vi "ScanDelay_FTIR.vi"() -> ()   [LabVIEW 2021]
uses:
  ScanDelay/Control_scanDelayWorkflow.ctl
  C:/Users/mnopl/Desktop/Software/LabVIEW/PRISM Scanning/Thorlabs.MotionControl.Controls.dll
  Thorlabs.MotionControl.Controls.dll
panel:
  in  "Cancel\nacquisition":bool
  in  "SerialNumber Flipper":string="37005305"
  in  "FilterFlipperControl":refnum<k24>(container)
  out "Spectrum stored":bool=TRUE
  out "Reference stored":bool=TRUE
  out "Normalized spectrum (phase)":T1(graph)={"Output spectrum"=[1102.5289175333148, 1103.2115979776079, 1103.894278421901, 1104.576958866194, 1105.259639310487, 1105.94231975478, 1106.6250001990732, 1107.3076806433662, 1107.9903610876595, 1108.6730415319525, 1109.3557219762456, 1110.0384024205387, 1110.7210828648317, 1111.4037633091248, 1112.0864437534178, 1112.7691241977109, 1113.451804642004, 1114.134485086297, 1114.81716553059, 1115.499845974883, 1116.1825264191764, 1116.8652068634694, 1117.5478873077625, 1118.2305677520555, 1118.9132481963486, 1119.5959286406417, 1120.2786090849347, 1120.9612895292278, 1121.6439699735208, 1122.3266504178139, 1123.009330862107, 1123.6920113064, 1124.3746917506933, 1125.0573721949863, 1125.7400526392794, 1126.4227330835724, 1127.1054135278655, 1127.7880939721585, 1128.4707744164516, 1129.1534548607447, 1129.8361353050377, 1130.5188157493308, 1131.2014961936238, 1131.8841766379169, 1132.5668570822102, 1133.2495375265032, 1133.9322179707963, 1134.6148984150893, 1135.2975788593824, 1135.9802593036754, 1136.6629397479685, 1137.3456201922615, 1138.0283006365546, 1138.7109810808477, 1139.3936615251407, 1140.0763419694338, 1140.759022413727, 1141.44170285802, 1142.1243833023132, 1142.8070637466062, 1143.4897441908993, 1144.1724246351923, 1144.8551050794854, 1145.5377855237784, 1146.2204659680715, 1146.9031464123645, 1147.5858268566576, 1148.2685073009507, 1148.951187745244, 1149.633868189537, 1150.31654863383, 1150.999229078123, 1151.6819095224162, 1152.3645899667092, 1153.0472704110023, 1153.7299508552953, 1154.4126312995884, 1155.0953117438814, 1155.7779921881745, 1156.4606726324675, 1157.1433530767608, 1157.826033521054, 1158.508713965347, 1159.19139440964, 1159.874074853933, 1160.556755298226, 1161.2394357425192, 1161.9221161868122, 1162.6047966311053, 1163.2874770753983, 1163.9701575196914, 1164.6528379639844, 1165.3355184082777, 1166.0181988525708, 1166.7008792968638, 1167.383559741157, 1168.06624018545, 1168.748920629743, 1169.431601074036, 1170.114281518329, 1170.7969619626222, 1171.4796424069152, 1172.1623228512083, 1172.8450032955013, 1173.5276837397946, 1174.2103641840877, 1174.8930446283807, 1175.5757250726738, 1176.2584055169668, 1176.94108596126], "Output spectrum"=[-1.328981625574806, -1.3297156380454427, -1.332925494608056, -1.3383669398670515, -1.3490986679786652, -1.3620665887791494, -1.3728322840821798, -1.3808051789599451, -1.38268785735066, -1.383454007683691, -1.3867362370563832, -1.392628994922722, -1.4079022417461098, -1.4232661538457454, -1.4254793325337713, -1.4234088794856259, -1.4261421511209245, -1.4345438849308945, -1.450738970302403, -1.4651556417192133, -1.472033577259217, -1.4765650658678406, -1.4767899466709609, -1.4779591915412682, -1.4864306235316898, -1.4967145833357045, -1.509311752447231, -1.5200946146126175, -1.5203325079241412, -1.518823068339795, -1.5221051369918865, -1.5289919543416084, -1.5443021693708103, -1.5596522358123068, -1.564563007819482, -1.564695009899656, -1.563485351619463, -1.564979237220899, -1.575817473163252, -1.5890558529666865, -1.598676891266045, -1.6047391447914532, -1.6037521530971257, -1.6021261032252092, -1.6080019905637195, -1.6176268726411671, -1.6308671920818638, -1.6420882814095819, -1.641366971284346, -1.6377105789186341, -1.6370525992687766, -1.6391413606802254, -1.6515063645518546, -1.6657201783289788, -1.6701214238463176, -1.6692686137411459, -1.664673373679217, -1.662735930327408, -1.6725089834242368, -1.6846208268448783, -1.6936098642043782, -1.6989794868515014, -1.6946893180335745, -1.6887570609947458, -1.6897142609229832, -1.6962784013144874, -1.7104316701396314, -1.7219554489591749, -1.7205768313097645, -1.716071748236028, -1.7122923695362096, -1.71258756824989, -1.7254368375091567, -1.7398505346411333, -1.74608798471659, -1.7471789380119624, -1.740606874293851, -1.7349037247161565, -1.7402490589291773, -1.7516392441731288, -1.7671122393723413, -1.7758636915304795, -1.7693645101770739, -1.7643499082781715, -1.7637118229070248, -1.765350147635751, -1.7796219339063313, -1.7937296960608236, -1.7953854575566122, -1.7914716614824544, -1.7856026813204544, -1.784818380975335, -1.7962387728445355, -1.812386692062692, -1.8233317957340986, -1.8247979168699975, -1.8161391987680926, -1.8112956667262592, -1.8161667026018287, -1.8247366793368631, -1.8389102094421166, -1.8495163568361097, -1.8449801698590533, -1.8376790464210524, -1.8356629006103997, -1.8413241156179243, -1.860416535366724, -1.8782177477731439, -1.881203280417375, -1.8755210713733286]}
  out "Normalized spectrum (amplitude)":T1(graph)={"Output spectrum"=[1102.5289175333148, 1103.2115979776079, 1103.894278421901, 1104.576958866194, 1105.259639310487, 1105.94231975478, 1106.6250001990732, 1107.3076806433662, 1107.9903610876595, 1108.6730415319525, 1109.3557219762456, 1110.0384024205387, 1110.7210828648317, 1111.4037633091248, 1112.0864437534178, 1112.7691241977109, 1113.451804642004, 1114.134485086297, 1114.81716553059, 1115.499845974883, 1116.1825264191764, 1116.8652068634694, 1117.5478873077625, 1118.2305677520555, 1118.9132481963486, 1119.5959286406417, 1120.2786090849347, 1120.9612895292278, 1121.6439699735208, 1122.3266504178139, 1123.009330862107, 1123.6920113064, 1124.3746917506933, 1125.0573721949863, 1125.7400526392794, 1126.4227330835724, 1127.1054135278655, 1127.7880939721585, 1128.4707744164516, 1129.1534548607447, 1129.8361353050377, 1130.5188157493308, 1131.2014961936238, 1131.8841766379169, 1132.5668570822102, 1133.2495375265032, 1133.9322179707963, 1134.6148984150893, 1135.2975788593824, 1135.9802593036754, 1136.6629397479685, 1137.3456201922615, 1138.0283006365546, 1138.7109810808477, 1139.3936615251407, 1140.0763419694338, 1140.759022413727, 1141.44170285802, 1142.1243833023132, 1142.8070637466062, 1143.4897441908993, 1144.1724246351923, 1144.8551050794854, 1145.5377855237784, 1146.2204659680715, 1146.9031464123645, 1147.5858268566576, 1148.2685073009507, 1148.951187745244, 1149.633868189537, 1150.31654863383, 1150.999229078123, 1151.6819095224162, 1152.3645899667092, 1153.0472704110023, 1153.7299508552953, 1154.4126312995884, 1155.0953117438814, 1155.7779921881745, 1156.4606726324675, 1157.1433530767608, 1157.826033521054, 1158.508713965347, 1159.19139440964, 1159.874074853933, 1160.556755298226, 1161.2394357425192, 1161.9221161868122, 1162.6047966311053, 1163.2874770753983, 1163.9701575196914, 1164.6528379639844, 1165.3355184082777, 1166.0181988525708, 1166.7008792968638, 1167.383559741157, 1168.06624018545, 1168.748920629743, 1169.431601074036, 1170.114281518329, 1170.7969619626222, 1171.4796424069152, 1172.1623228512083, 1172.8450032955013, 1173.5276837397946, 1174.2103641840877, 1174.8930446283807, 1175.5757250726738, 1176.2584055169668, 1176.94108596126], "Output spectrum"=[1.0873076708633411, 1.08394867428729, 1.0888562107920463, 1.0969307314805181, 1.102998120422263, 1.107136071600766, 1.1035642445072202, 1.0961034542227839, 1.094872735773217, 1.1010416062836017, 1.1106100405553267, 1.115942213485196, 1.1130278245062957, 1.1072973234979273, 1.102059722167887, 1.098186618808356, 1.1015816281752067, 1.108746473864395, 1.111756741956775, 1.1105953151312484, 1.1032227061156759, 1.0952300942782656, 1.0958494687443006, 1.1007057231621713, 1.106295224941442, 1.1104780174250957, 1.1057667534821705, 1.0964576694777417, 1.0904090869006036, 1.088459311408212, 1.0942598558444103, 1.1012239259596472, 1.0993344675621843, 1.092466822796523, 1.0835822296721949, 1.0759964933630453, 1.0774338793339753, 1.0829818692266655, 1.085123774157756, 1.0835731005973663, 1.0747228497785382, 1.0629565097932145, 1.0579906286730316, 1.058422967601046, 1.0630212715521237, 1.0675638836007573, 1.0625734863702079, 1.0529318841119182, 1.0449994916681102, 1.0391477625279653, 1.0421567088004438, 1.0486532412237262, 1.0477398261213626, 1.0417732985786687, 1.03113814399867, 1.0200979633688834, 1.0182230978827198, 1.022584163574115, 1.0286739828363953, 1.032026518895644, 1.0242044127425998, 1.011323536655613, 1.0049354451214019, 1.0053102459549301, 1.011993306853234, 1.0193524696815321, 1.0176245623256048, 1.0098015162659275, 0.9995985179330682, 0.9919293607652324, 0.995810871440088, 1.0045616890791953, 1.0093618831764462, 1.008860094407166, 0.9990320036845148, 0.9874622731652223, 0.9856201758039206, 0.9912449764462133, 0.9997370337275218, 1.0041657589490753, 0.9979424163566785, 0.9878008483696279, 0.9797038935662515, 0.9774024796092163, 0.9873954031846796, 0.9975940631540408, 0.996754666997269, 0.990809571391422, 0.9797449519284779, 0.9700271866511746, 0.9728145275232338, 0.9828560719840351, 0.9916163639682382, 0.9946994569688331, 0.9866468392828865, 0.9740403779039128, 0.9670830091995587, 0.9689347920073221, 0.9807941187046116, 0.9896212414408725, 0.9843156725932524, 0.9762091225257215, 0.969940310795789, 0.9659022733566544, 0.9737200015171775, 0.9861338055781489, 0.988751689371605, 0.983147618233142, 0.9731806985492104, 0.9653668962641432]}
  in  "Store as reference":bool
  out "Python alpha rep path":path=path "C:/Users/mnopl/Desktop/Software/python/alpha/rep.py"
  out "Activity status":string="Awaiting command"
  out "Acquisition status":string="Ready to acquire spectrum"
  in  "Save spectrum to path":path
  in  "Load reference":bool
  in  "Load reference from path":path
  in  "Load spectrum from path":path
  in  "Apply spectral\nenvelope":bool=TRUE
  out "Binned interferogram":cluster{"X":dbl, "Y":dbl}[](graph)
  out "Reference Spectra":dbl[][](array[numeric])
  out "Analyte Spectra":dbl[][](array[numeric])
  out "Python error: spectrum acquisition":errorcluster={"status"=TRUE, "code"=1666, "source"="Python Node in ScanDelay_FTIR.vi"}
  out "Python scandelay path":path=path "C:/Users/mnopl/Desktop/Software/LabVIEW/ScanDelay/scandelay.py"
  in  "Time per\nacquisition (s)":dbl=8.5
  in  "Sampling rate":dbl=250000.0
  in  "Delay calibration\n          factor":dbl=2.403 format="%_6g"
  in  "Acquisitions per\ninterferogram":i32=1
  in  "Bins per\ninterferogram":i32=30000
  in  "Subtract\nphase slope\n (2pi * dx)":dbl=-0.001
  out "Python error: DAQ acquisition":errorcluster
  out "# Accumulated":i32=4
  in  "Accumulate to #":i32=4
  out "Latest alpha cmd":string="@rep load 9"
  in  "Replicate alpha\non accumulate?":bool
  out "Accumulated spectrum (amplitude)":T1(graph)
  out "Accumulated spectrum (phase)":T1(graph)
  out "Acquisition cycle":dbl[][](graph)
  out "% averaged":dbl=100.0
  in  "Pause\nacquisition":bool
  in  "Halt program":bool
  out "Python error: activity loop":errorcluster
  in  "Load spectrum":bool
  in  "Save spectrum":bool
  in  "Normalize spectrum":bool
  in  "Acquire spectrum":bool
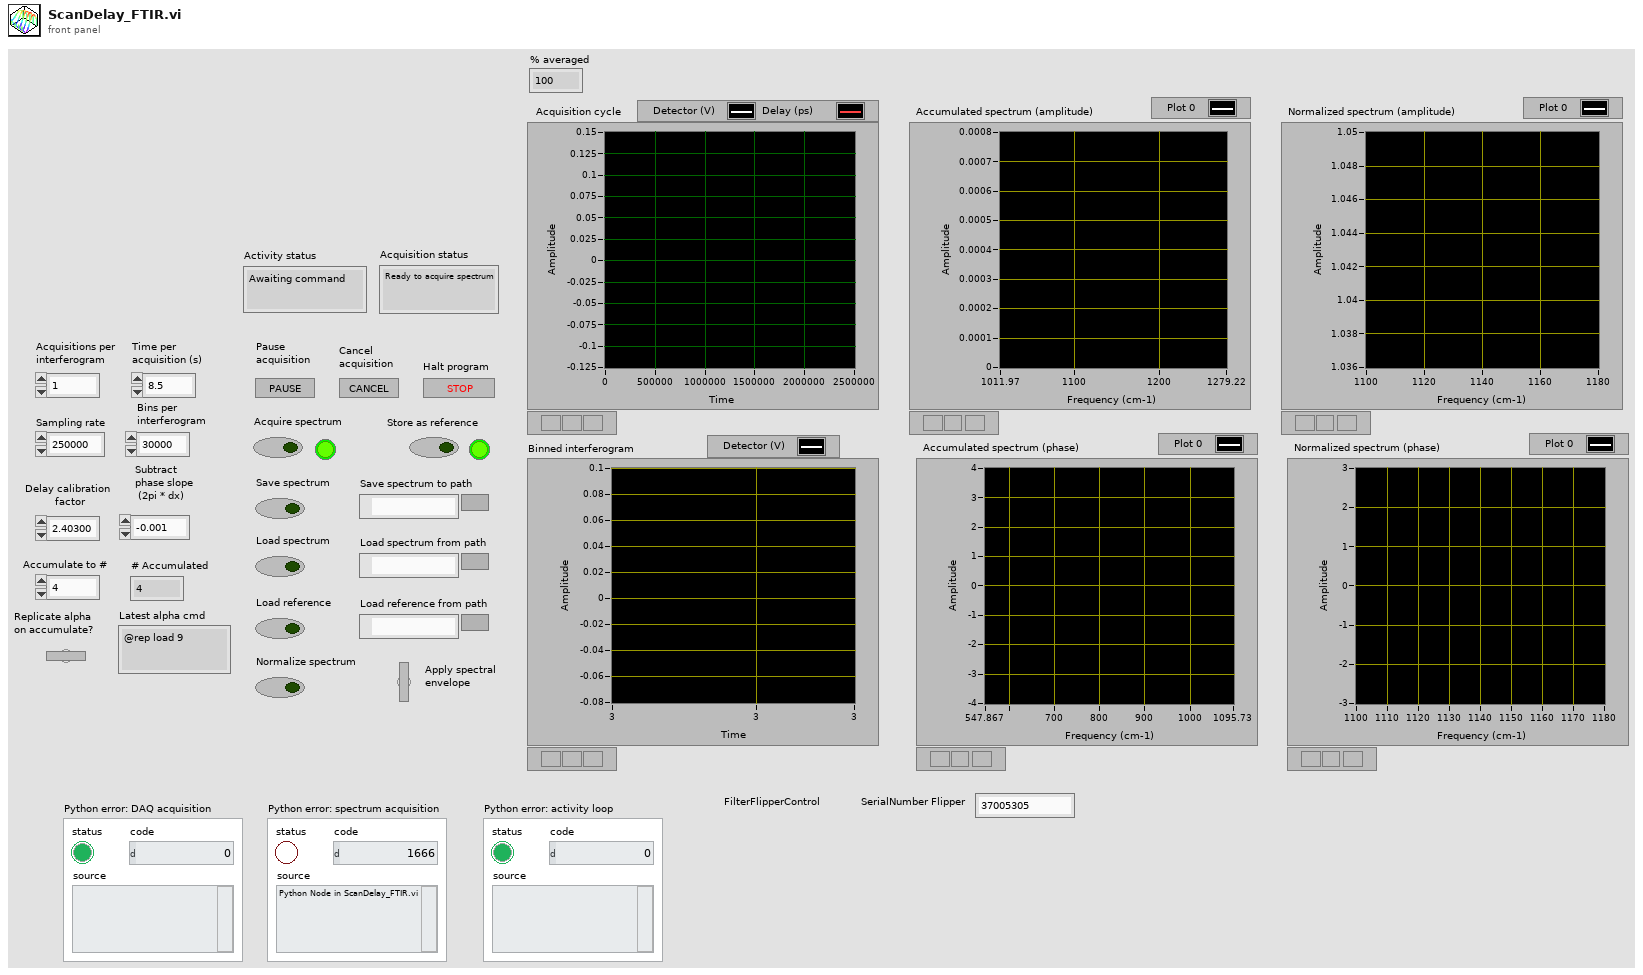
[diagram p1: front panel]
types:
  T1 = cluster{"Output spectrum":dbl[], "Output spectrum":dbl[]}
  T2 = typedef "Control_scanDelayWorkflow.ctl" = enum16{"Initialize", "Sit Idle", "Load Spectrum", "Store reference", "Save Spectrum", "Load reference", "Check Reference", "Check Spectrum", "Normalize Spectrum", "Done"}
  T3 = cluster{"Analyte Spectra":dbl[], "Analyte Spectra":dbl[]}
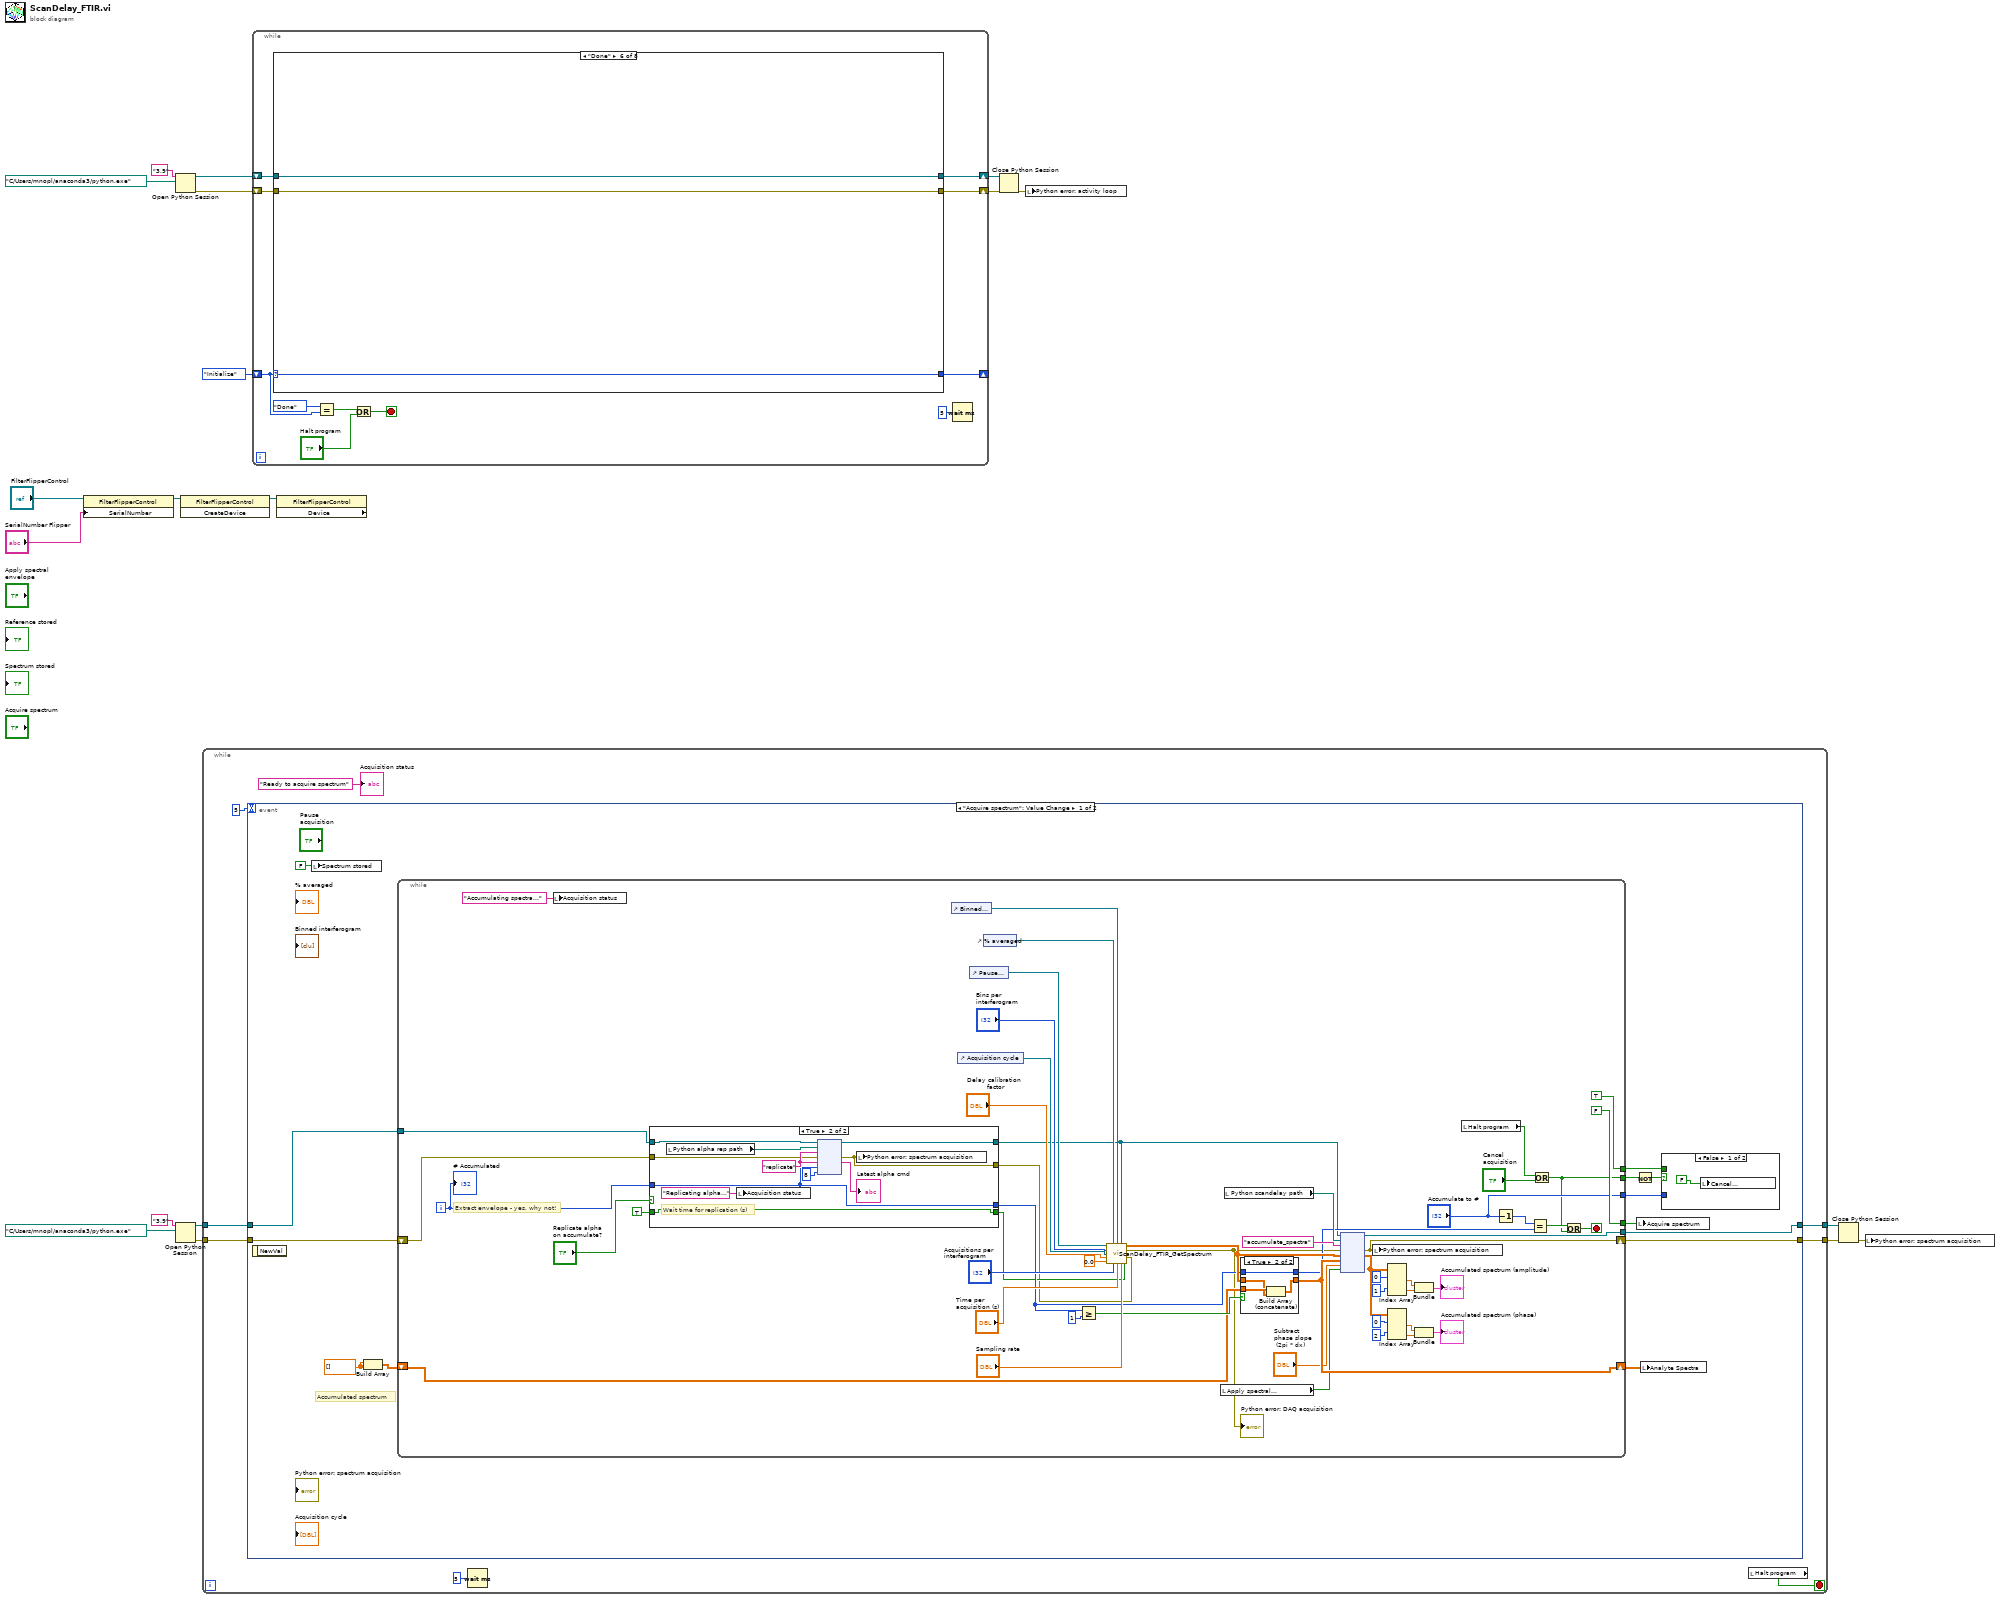
[diagram p0: block diagram]
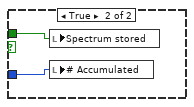
[diagram p2: hidden frame]
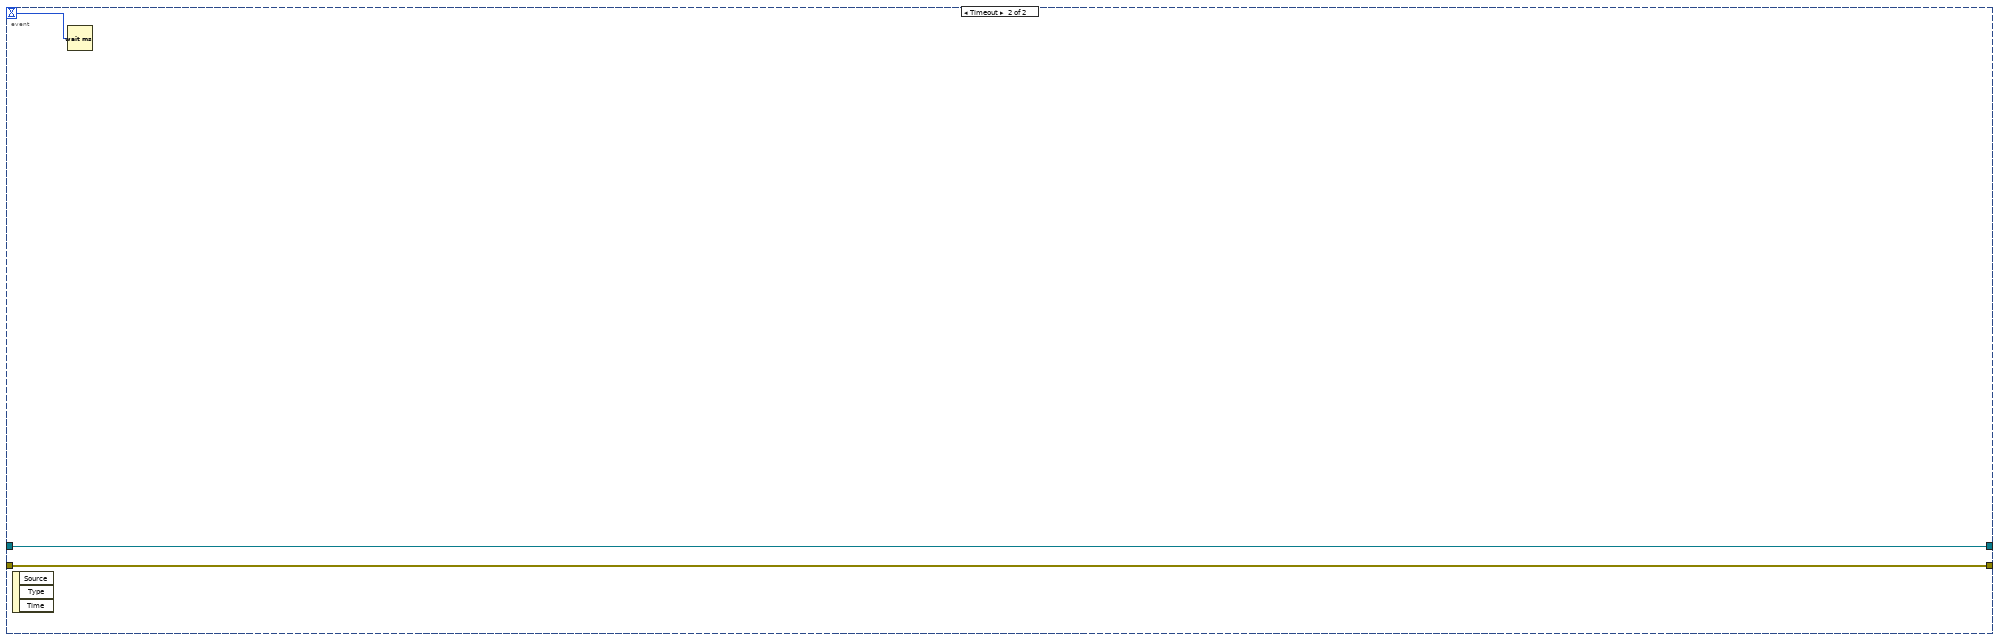
[diagram p5: hidden frame]
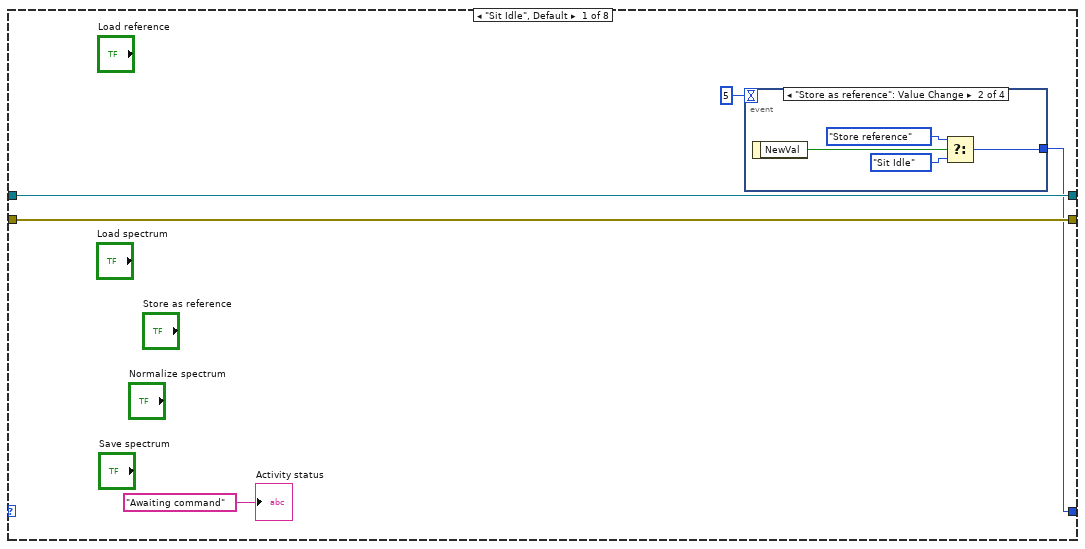
[diagram p6: hidden frame]
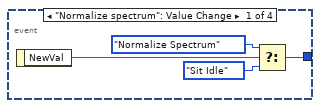
[diagram p7: hidden frame]
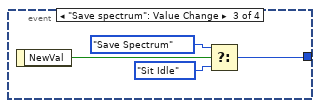
[diagram p8: hidden frame]
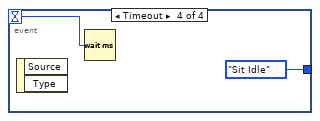
[diagram p9: hidden frame]
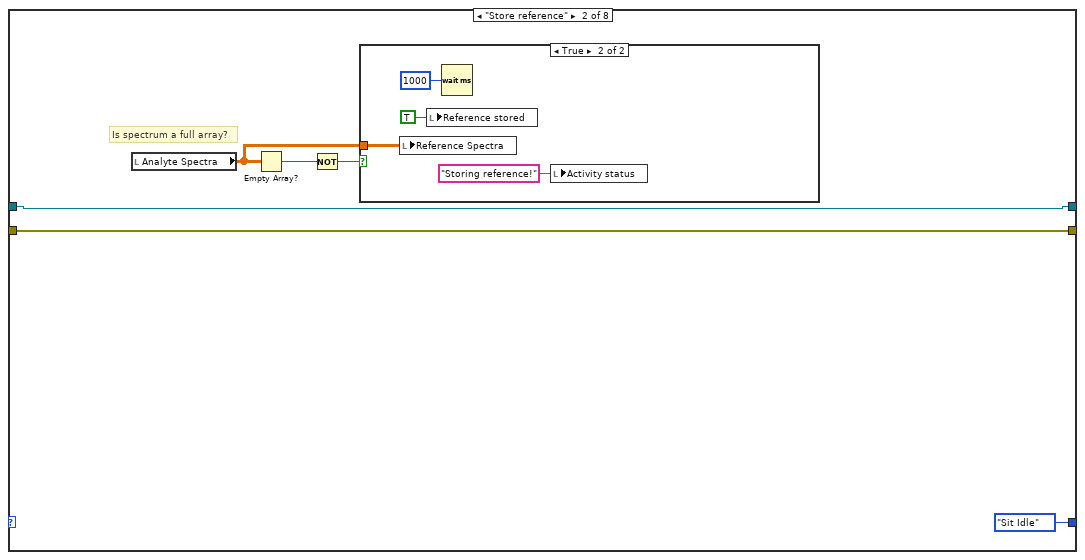
[diagram p10: hidden frame]
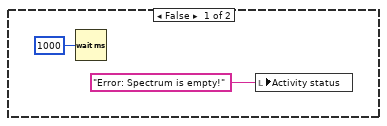
[diagram p11: hidden frame]
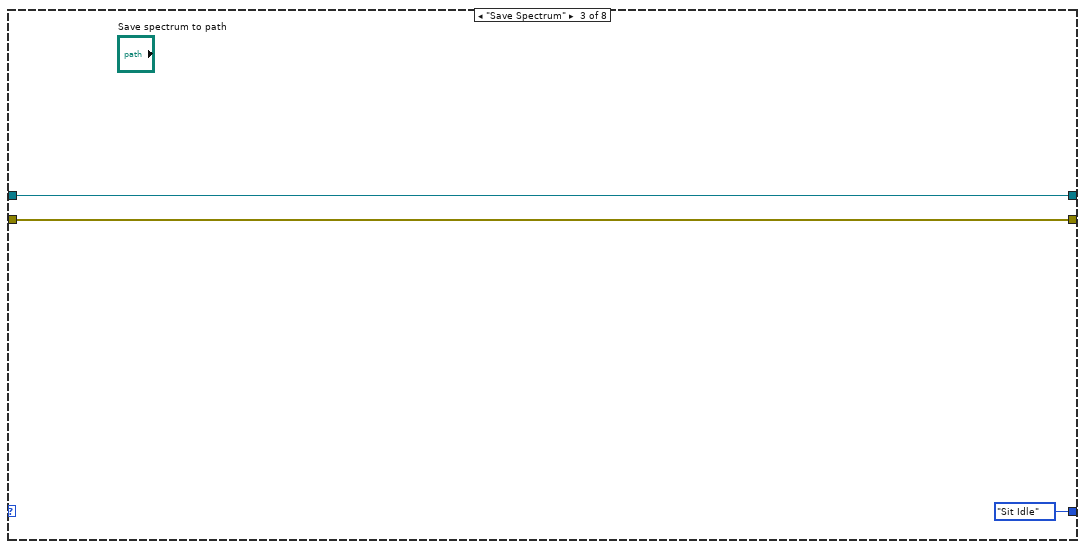
[diagram p12: hidden frame]
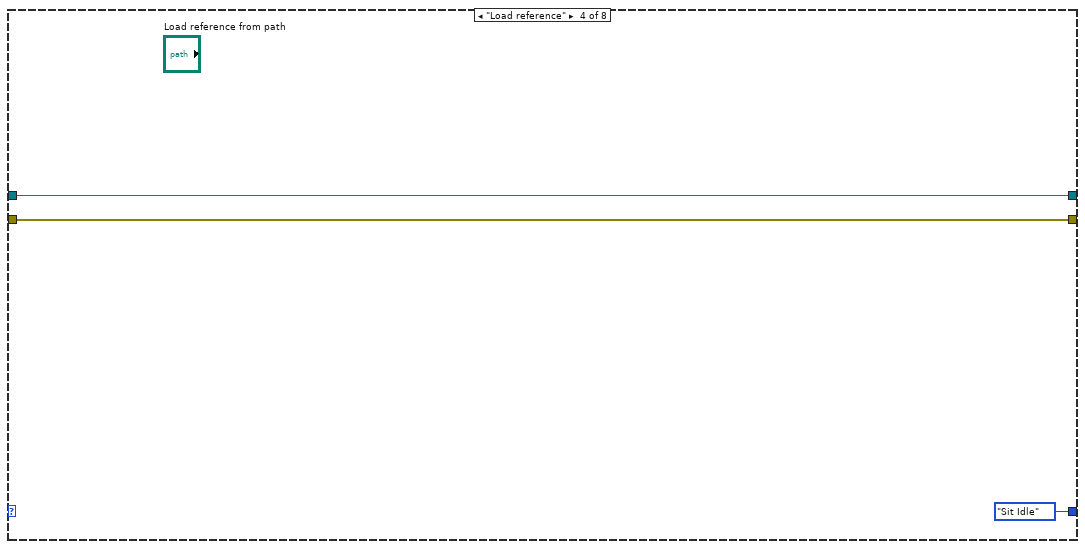
[diagram p13: hidden frame]
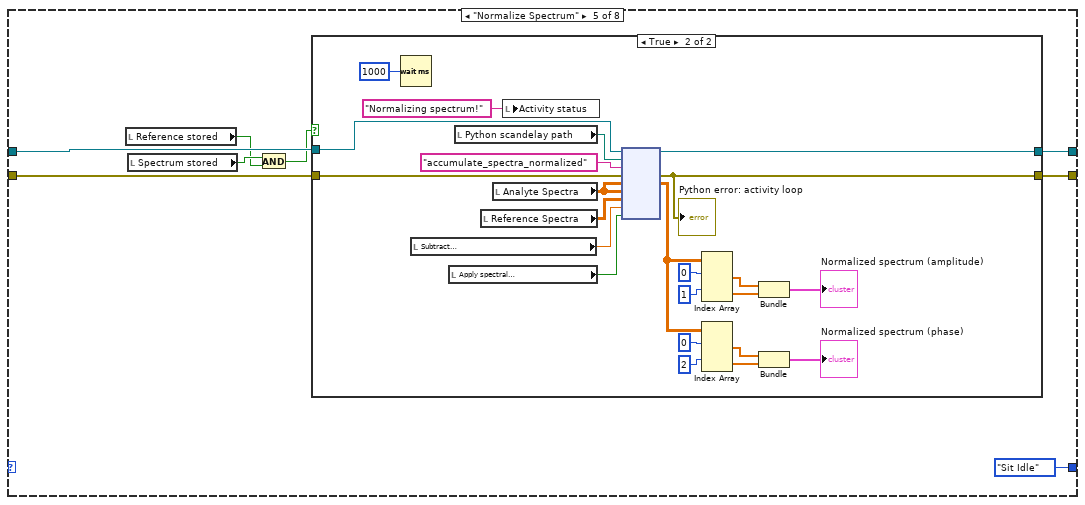
[diagram p14: hidden frame]
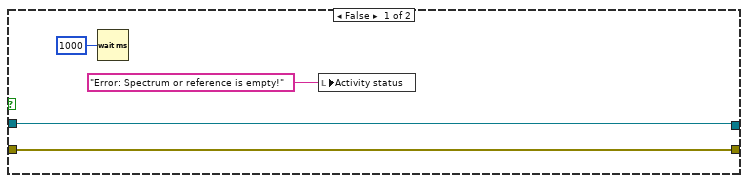
[diagram p15: hidden frame]
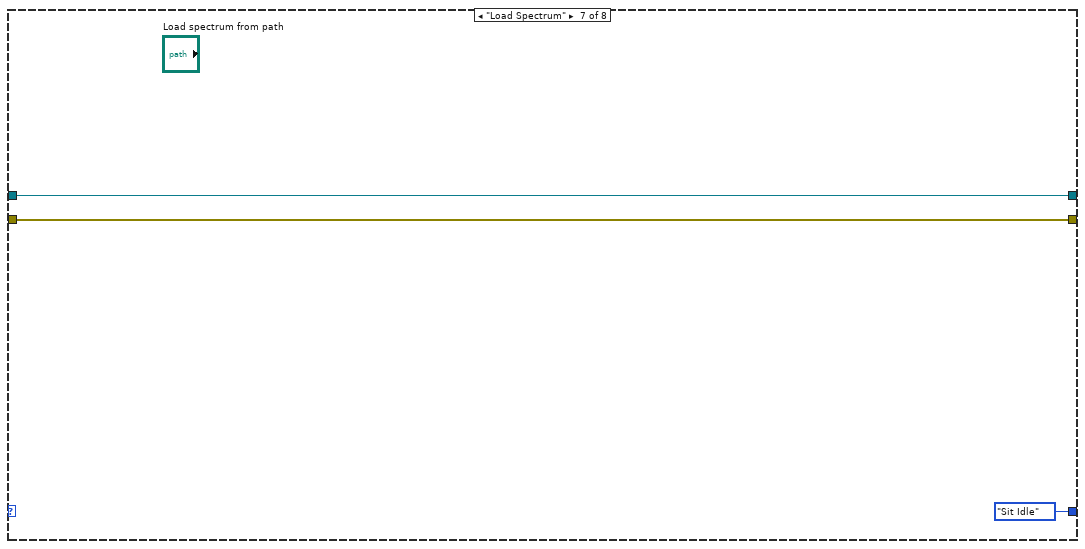
[diagram p16: hidden frame]
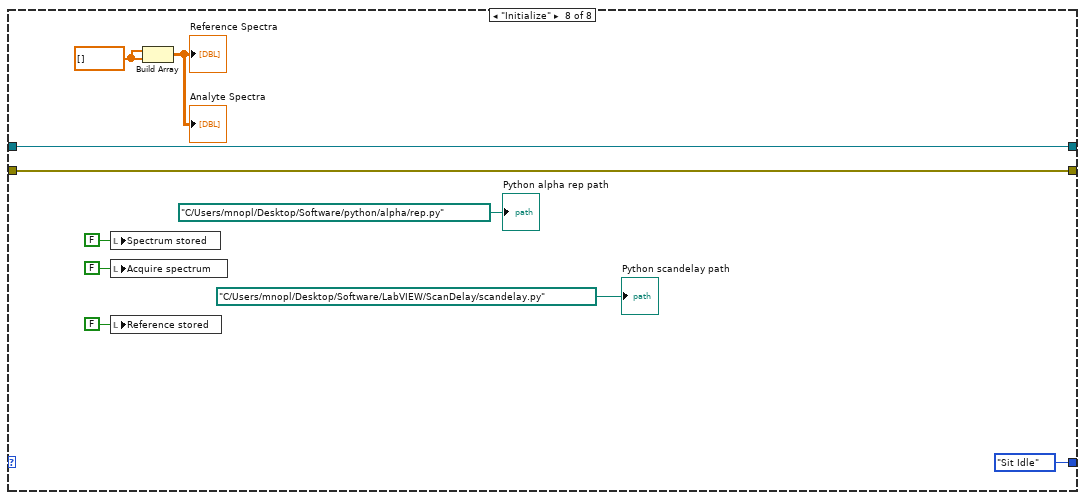
[diagram p17: hidden frame]
diagram:
  n1 = property class="FilterFlipperControl"(reference="FilterFlipperControl", "SerialNumber"="SerialNumber Flipper") -> (reference out=w2:refnum<k24>)  [unwired: 1 in, 1 out]
  n2 = Open Python Session(python version="3.9", python path=path "C:/Users/mnopl/anaconda3/python.exe") -> (session out=w8:refnum<k35>, error out=w7:errorcluster)  [unwired: 1 in]
  n3 = Open Python Session(python version="3.9", python path=path "C:/Users/mnopl/anaconda3/python.exe") -> (session out=w12:refnum<k35>, error out=w11:errorcluster)  [unwired: 1 in]
  n4 = invoke class="FilterFlipperControl" method="CreateDevice"(reference=w2) -> (reference out=w1:refnum<k24>)  [unwired: 2 in, 2 out]
  n5 = while {
    tunnel: w12 -> [w26]
    tunnel: w11 -> [w25]
    tunnel: [w24] -> w10
    tunnel: [w23] -> w9
    stop <- w27 stop-if-true
    n6 = event shown="[0] \"Acquire spectrum\": Value Change" {
      selector: _ -> [_ _]
      dyn-events: _ -> [_ _]
      timeout: 5 -> [_ w120]
      tunnel: w26 -> [w37 w118]
      tunnel: w25 -> [w36 w119]
      tunnel: [w35 w118] -> w24
      tunnel: [w33 w119] -> w23
      event "Acquire spectrum": Value Change {
        w39 = dbl[] []
        # "Accumulated spectrum"
        n7 = event-data() -> ()  [unwired: 1 in, 1 out]
        n8 = local write "Spectrum stored"(FALSE) -> ()
        n9 = Build Array(w39, w39) -> (w40:dbl[][])
        n10 = while {
          shift-right: [w74] -> w38
          shift-left: w40 -> [w87]
          tunnel: [w55] -> w35
          tunnel: w37 -> [w58]
          tunnel: [FALSE] -> w34
          shift-right: [w49] -> w33
          shift-left: w36 -> [w57]
          tunnel: [TRUE] -> w31
          tunnel: ["Accumulate to #"] -> w30
          tunnel: [w44] -> w28
          i -> [w51]
          stop <- w61 stop-if-true
          # "Extract envelope - yes, why not!"
          n11 = local write "Acquisition status"("Accumulating spectra...") -> ()
          n12 = case shown="True" "Replicate alpha\non accumulate?" {
            tunnel: w57 -> [w99 w108]
            tunnel: w58 -> [w100 w107]
            tunnel: [w100 w106] -> w46
            tunnel: [w99 w101] -> w48
            tunnel: w51 -> [w98 w103]
            tunnel: [w98 w103] -> w56
            tunnel: TRUE -> [w97 w102]
            tunnel: [w97 w102] -> w53
            frame False {
            }
            frame True {
              w109 = "replicate"
              # "Wait time for replication (s)"
              n13 = local read "Python alpha rep path"() -> (w104:path)
              n14 = local write "Acquisition status"("Replicating alpha...") -> ()
              n15 = node(w107, w104, w109, w108, w109, w103, 8) -> (w106:refnum<k35>, w101:errorcluster, →"Latest alpha cmd":string)  [unwired: 2 in, 2 out]
              n16 = local write "Python error: spectrum acquisition"(w101) -> ()
            }
          }
          n17 = control-ref of="Binned interferogram"() -> (w76:refnum<vi>)
          n18 = control-ref of="Acquisition cycle"() -> (w96:refnum<vi>)
          n19 = control-ref of="Pause\nacquisition"() -> (w91:refnum<vi>)
          n20 = control-ref of="% averaged"() -> (w92:refnum<vi>)
          n21 = Greater Or Equal?(x=w56, y=1) -> (x >= y?=w89:bool)
          n22 = call "ScanDelay_FTIR_GetSpectrum.vi"("Acquire / Pause? External"=w91, "% averaged (external)"=w92, "Binned interferogram (external)"=w76, "Python refnum in"=w46, "N delays"="Bins per\ninterferogram", "Acquisition cycle (external)"=w96, "Delay calibration\n          factor"="Delay calibration\n          factor", "Python error in"=w48, "Subtract\ndelay (ps)"=0.0, "Acquisitions per interferogram"="Acquisitions per\ninterferogram", "Time per acquisition (s)"="Time per\nacquisition (s)", "Sampling rate"="Sampling rate", "Extract envelope"=w53) -> ("Output spectrum"=w69:dbl[][], "Python error"=w47:errorcluster)  [unwired: 1 in]
          "Python error: DAQ acquisition" <- w47
          n23 = local read "Apply spectral\nenvelope"() -> (w65:bool)
          n24 = local read "Python scandelay path"() -> (w67:path)
          n25 = case shown="True" w89 {
            tunnel: w69 -> [w113 w116]
            tunnel: w87 -> [_ w117]
            tunnel: [w113 w115] -> w74
            tunnel: w56 -> [w112 w114]
            tunnel: [w112 w114] -> w52
            frame False {
            }
            frame True {
              n26 = Build Array (concatenate)(w117, w116) -> (w115:dbl[][])
            }
          }
          n27 = node(w46, w67, "accumulate_spectra", w47, w69, w74, "Subtract\nphase slope\n (2pi * dx)", w65) -> (w55:refnum<k35>, w49:errorcluster, w68:dbl[][])  [unwired: 3 in, 2 out]
          n28 = local write "Python error: spectrum acquisition"(w49) -> ()
          n29 = Index Array(array=w68, index (row) #1=0, index (row) #2=1) -> (element #1=w83:dbl[], element #2=w82:dbl[])  [unwired: 2 in]
          n30 = Index Array(array=w68, index (row) #1=0, index (row) #2=2) -> (element #1=w79:dbl[], element #2=w78:dbl[])  [unwired: 2 in]
          n31 = Bundle("Output spectrum"=w83, "Output spectrum"=w82) -> (→"Accumulated spectrum (amplitude)":T1)  [unwired: 1 in]
          n32 = Bundle("Output spectrum"=w79, "Output spectrum"=w78) -> (→"Accumulated spectrum (phase)":T1)  [unwired: 1 in]
          n33 = local read "Halt program"() -> (w50:bool)
          n34 = Decrement(x="Accumulate to #") -> (x-1=w60:i32)
          n35 = Equal?(x=w60, y=w52) -> (x = y?=w70:bool)
          n36 = Or(x=w50, y="Cancel\nacquisition") -> (x .or. y?=w44:bool)
          n37 = Or(x=w70, y=w44) -> (x .or. y?=w61:bool)
          "# Accumulated" <- w51
        }
        n38 = Not(x=w28) -> (.not. x?=w29:bool)
        n39 = local write "Acquire spectrum"(w34) -> ()
        n40 = local write "Analyte Spectra"(w38) -> ()
        n41 = case shown="False" w29 {
          tunnel: w31 -> [_ w43]
          tunnel: w30 -> [_ w42]
          frame False {
            n42 = local write "Cancel\nacquisition"(FALSE) -> ()
          }
          frame True {
            n43 = local write "Spectrum stored"(w43) -> ()
            n44 = local write "# Accumulated"(w42) -> ()
          }
        }
      }
      event Timeout {
        n45 = event-data() -> ()  [unwired: 1 in, 3 out]
        n46 = Wait (ms)(milliseconds to wait=w120) -> ()  [unwired: 1 out]
      }
    }
    n47 = Wait (ms)(milliseconds to wait=5) -> ()  [unwired: 1 out]
    n48 = local read "Halt program"() -> (w27:bool)
    "Acquisition status" <- "Ready to acquire spectrum"
  }
  n49 = while {
    shift-right: [w123] -> _
    shift-left: Control_scanDelayWorkflow."Initialize" -> [w129]
    shift-right: [w130] -> w15
    shift-left: w7 -> [w121]
    shift-right: [w124] -> w16
    shift-left: w8 -> [w122]
    stop <- w127 stop-if-true
    n50 = case shown="\"Done\"" w129 {
      selector: w129 -> [_ _ _ _ _ w204 _ _]
      tunnel: [w135 w156 w165 w167 w172 w205 w208 w215] -> w130
      tunnel: w122 -> [w136 w155 w164 w168 w175 w206 w209 w216]
      tunnel: w121 -> [w135 w156 w165 w167 w174 w205 w208 w215]
      tunnel: [w136 w155 w164 w168 w173 w206 w209 w216] -> w124
      tunnel: [w134 Control_scanDelayWorkflow."Sit Idle" Control_scanDelayWorkflow."Sit Idle" Control_scanDelayWorkflow."Sit Idle" Control_scanDelayWorkflow."Sit Idle" w204 Control_scanDelayWorkflow."Sit Idle" Control_scanDelayWorkflow."Sit Idle"] -> w123
      frame "Sit Idle", Default {
        n51 = event shown="[1] \"Store as reference\": Value Change" {
          selector: _ -> [_ _ _ _]
          dyn-events: _ -> [_ _ _ _]
          timeout: 5 -> [_ _ _ w149]
          tunnel: [w137 w141 w145 Control_scanDelayWorkflow."Sit Idle"] -> w134
          event "Normalize spectrum": Value Change {
            n52 = event-data() -> ("NewVal"=w138:bool)  [unwired: 1 in]
            n53 = Select(t=Control_scanDelayWorkflow."Normalize Spectrum", s=w138, f=Control_scanDelayWorkflow."Sit Idle") -> (s? t:f=w137:T2)
          }
          event "Store as reference": Value Change {
            n54 = event-data() -> ("NewVal"=w144:bool)  [unwired: 1 in]
            n55 = Select(t=Control_scanDelayWorkflow."Store reference", s=w144, f=Control_scanDelayWorkflow."Sit Idle") -> (s? t:f=w141:T2)
          }
          event "Save spectrum": Value Change {
            n56 = event-data() -> ("NewVal"=w146:bool)  [unwired: 1 in]
            n57 = Select(t=Control_scanDelayWorkflow."Save Spectrum", s=w146, f=Control_scanDelayWorkflow."Sit Idle") -> (s? t:f=w145:T2)
          }
          event Timeout {
            n58 = event-data() -> ()  [unwired: 1 in, 2 out]
            n59 = Wait (ms)(milliseconds to wait=w149) -> ()  [unwired: 1 out]
          }
        }
        "Activity status" <- "Awaiting command"
      }
      frame "Store reference" {
        # "Is spectrum a full array?"
        n60 = local read "Analyte Spectra"() -> (w151:dbl[][])
        n61 = Empty Array?(array=w151) -> (empty?=w153:bool)
        n62 = Not(x=w153) -> (.not. x?=w152:bool)
        n63 = case shown="True" w152 {
          tunnel: w151 -> [_ w161]
          frame False {
            n64 = Wait (ms)(milliseconds to wait=1000) -> ()  [unwired: 1 out]
            n65 = local write "Activity status"("Error: Spectrum is empty!") -> ()
          }
          frame True {
            n66 = local write "Reference Spectra"(w161) -> ()
            n67 = local write "Reference stored"(TRUE) -> ()
            n68 = Wait (ms)(milliseconds to wait=1000) -> ()  [unwired: 1 out]
            n69 = local write "Activity status"("Storing reference!") -> ()
          }
        }
      }
      frame "Save Spectrum" {
      }
      frame "Load reference" {
      }
      frame "Normalize Spectrum" {
        n70 = local read "Reference stored"() -> (w170:bool)
        n71 = local read "Spectrum stored"() -> (w171:bool)
        n72 = And(x=w171, y=w170) -> (x .and. y?=w169:bool)
        n73 = case shown="True" w169 {
          tunnel: w175 -> [w178 w202]
          tunnel: w174 -> [w177 w201]
          tunnel: [w178 w200] -> w173
          tunnel: [w177 w181] -> w172
          frame False {
            n74 = Wait (ms)(milliseconds to wait=1000) -> ()  [unwired: 1 out]
            n75 = local write "Activity status"("Error: Spectrum or reference is empty!") -> ()
          }
          frame True {
            n76 = Wait (ms)(milliseconds to wait=1000) -> ()  [unwired: 1 out]
            n77 = local read "Subtract\nphase slope\n (2pi * dx)"() -> (w197:dbl)
            n78 = local read "Apply spectral\nenvelope"() -> (w196:bool)
            n79 = local read "Python scandelay path"() -> (w199:path)
            n80 = local read "Reference Spectra"() -> (w183:dbl[][])
            n81 = local read "Analyte Spectra"() -> (w182:dbl[][])
            n82 = local write "Activity status"("Normalizing spectrum!") -> ()
            n83 = node(w202, w199, "accumulate_spectra_normalized", w201, w182, w182, w183, w197, w196) -> (w200:refnum<k35>, w181:errorcluster, w185:dbl[][])  [unwired: 4 in, 2 out]
            "Python error: activity loop" <- w181
            n84 = Index Array(array=w185, index (row) #1=0, index (row) #2=1) -> (element #1=w193:dbl[], element #2=w192:dbl[])  [unwired: 2 in]
            n85 = Index Array(array=w185, index (row) #1=0, index (row) #2=2) -> (element #1=w189:dbl[], element #2=w188:dbl[])  [unwired: 2 in]
            n86 = Bundle("Analyte Spectra"=w193, "Analyte Spectra"=w192) -> (→"Normalized spectrum (amplitude)":T3)  [unwired: 1 in]
            n87 = Bundle("Analyte Spectra"=w189, "Analyte Spectra"=w188) -> (→"Normalized spectrum (phase)":T3)  [unwired: 1 in]
          }
        }
      }
      frame "Done" {
      }
      frame "Load Spectrum" {
      }
      frame "Initialize" {
        w217 = dbl[] []
        n88 = local write "Spectrum stored"(FALSE) -> ()
        n89 = local write "Acquire spectrum"(FALSE) -> ()
        n90 = local write "Reference stored"(FALSE) -> ()
        n91 = Build Array(w217, w217) -> (→"Analyte Spectra" →"Reference Spectra":dbl[][])
        "Python scandelay path" <- path "C:/Users/mnopl/Desktop/Software/LabVIEW/ScanDelay/scandelay.py"
        "Python alpha rep path" <- path "C:/Users/mnopl/Desktop/Software/python/alpha/rep.py"
      }
    }
    n92 = Equal?(x=Control_scanDelayWorkflow."Done", y=w129) -> (x = y?=w125:bool)
    n93 = Or(x=w125, y="Halt program") -> (x .or. y?=w127:bool)
    n94 = Wait (ms)(milliseconds to wait=5) -> ()  [unwired: 1 out]
  }
  n95 = property class="FilterFlipperControl" props=["Device"](reference=w1) -> ()  [unwired: 1 in, 3 out]
  n96 = Close Python Session(session in=w16, error in=w15) -> (11:w5:errorcluster)
  n97 = local write "Python error: activity loop"(w5) -> ()
  n98 = Close Python Session(session in=w10, error in=w9) -> (11:w6:errorcluster)
  n99 = local write "Python error: spectrum acquisition"(w6) -> ()
